vi "ADIS16448 IMU Example.vi"() -> ()   [LabVIEW 2015]
doc: "SimpleGyro Example\n\nThis example shows how to use a SimpleGyro sensor connected to the SPI port on the RoboRIO.\n\nThis example expects a USB cable connected from your development PC to the Type B USB Jack (next to the power input) on the roboRIO."
uses:
  <vilib>/Rock Robotics/SystemInterfaces/spilib/spi_bus.ctl
  ADI MXP IMU/FRC_ADIS16448_IMU.lvlib
panel:
  out "IMU Angle Delta":cluster{"X":dbl, "Y":dbl, "Z":dbl} {"X" scale=-180.0..180.0; "Y" scale=-180.0..180.0; "Z" scale=-180.0..180.0}
  out "IMU AHRS":cluster{"Pitch":dbl, "Roll":dbl, "Yaw":dbl} {"Roll" scale=-180.0..180.0; "Pitch" scale=-90.0..90.0}
  out "IMU Data Out":T1 {"X Accel (g)" format="%#_3g"; "Y Accel (g)" format="%#_3g"; "Z Accel (g)" format="%#_3g"}
  in  "AHRS Algorithm":enum16{"Complementary", "Madgwick"}(ring)
  in  "AHRS Yaw Axis":enum16{"X", "Y", "Z"}(ring)=enum."Z"
  out "Sensor Ready?":bool
  out "IMU AHRS":cluster{"Pitch":dbl, "Roll":dbl, "Yaw":dbl}
  out "IMU Angle Delta":cluster{"X":dbl, "Y":dbl, "Z":dbl}
  in  "Reset Deltas?":bool
  out "Device Found?":bool
  in  "stop":bool
  # "FRC Analog Devices ADIS16448 IMU Example"
  # "Raw IMU Output Data"
  # "FRC ADI MXP Placement"
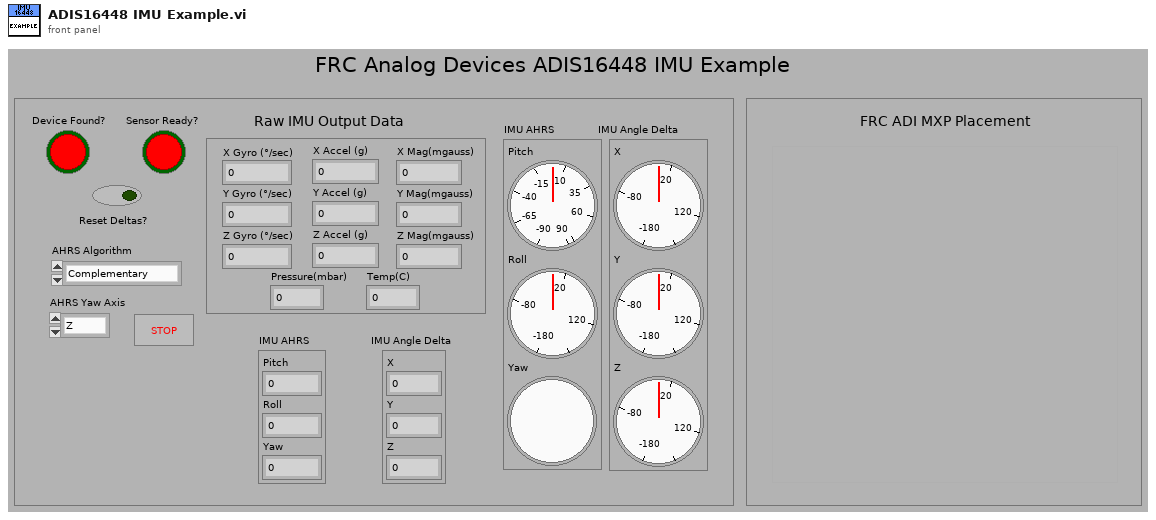
[diagram p1: front panel]
types:
  T1 = cluster{"X Gyro (°/sec)":dbl, "Y Gyro (°/sec)":dbl, "Z Gyro (°/sec)":dbl, "X Accel (g)":dbl, "Y Accel (g)":dbl, "Z Accel (g)":dbl, "X Mag(mgauss)":dbl, "Y Mag(mgauss)":dbl, "Z Mag(mgauss)":dbl, "Pressure(mbar)":dbl, "Temp(C)":dbl}
  T2 = typedef "spi_bus.ctl" = enum16{"SPI On-Board, CS0", "SPI On-Board, CS1", "SPI On-Board, CS2", "SPI On-Board, CS3", "SPI MXP", "Invalid"}
  T3 = typedef "FRC_ADIS16448_IMU.lvlib/WPI_IMU_ADIS16448_InterruptDevRef.ctl" = cluster{"ADI IMU DevRef":T4, "InterruptRef":T5}
  T4 = typedef "FRC_ADIS16448_IMU.lvlib/WPI_IMU_ADIS16448_IMUDevRef.ctl" = cluster{"DevStatus":errorcluster, "Handle":i32, "SPI Bus":T2, "Device Found":bool, "Device Ready":bool, "Yaw Axis":enum16{"X", "Y", "Z"}, "AHRS Algorithm":enum16{"Complementary", "Madgwick"}, "Serial":u16, "Lot ID 2":u16, "Lot ID 1":u16, "Product ID":u16}
  T5 = typedef "WPI_InterruptRef.ctl" = cluster{"DevStatus":errorcluster, "InterruptIndex":T6}
  T6 = typedef "FPGA_InterruptIndex.ctl" = enum8{"0", "1", "2", "3", "4", "5", "6", "7", "Invalid"}
  T7 = cluster{"X Angle":dbl, "Y Angle":dbl, "Z Angle":dbl}
  T8 = cluster{"X Gyro":dbl, "Y Gyro":dbl, "Z Gyro":dbl, "X Accel":dbl, "Y Accel":dbl, "Z Accel":dbl, "X Mag":dbl, "Y Mag":dbl, "Z Mag":dbl, "Pressure":dbl, "Temp":dbl}
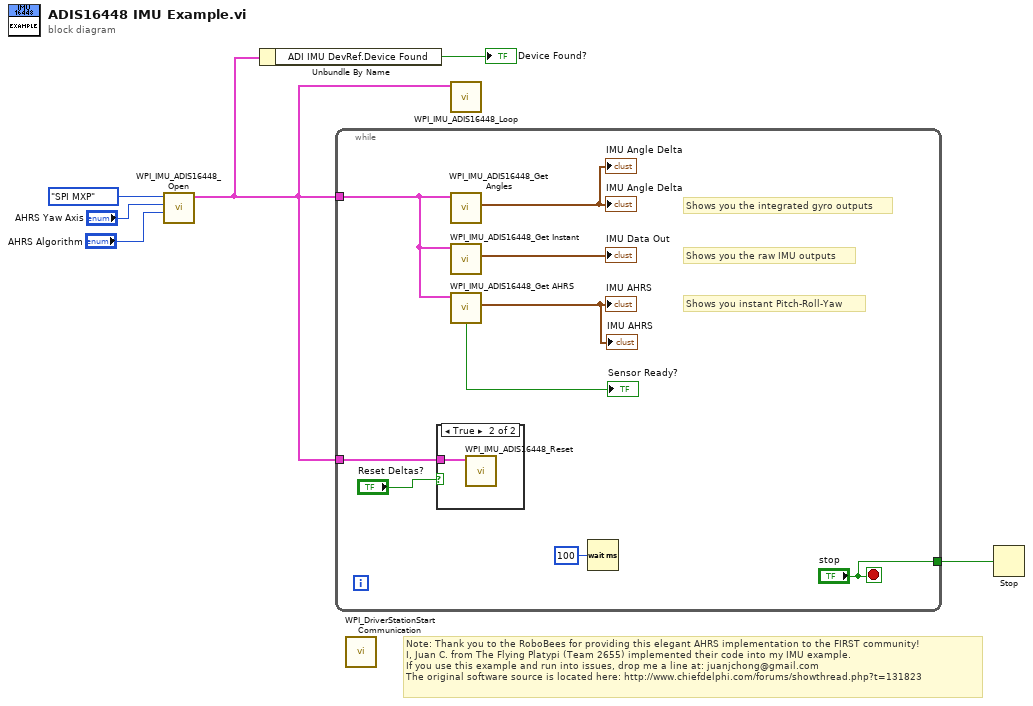
[diagram p0: block diagram]
diagram:
  # "Note: Thank you to the RoboBees for providing this elegant AHRS implementation to the FIRST community!\nI, Juan C. from The Flying Platypi (Team 2655) implemented their code into my IMU example.\nIf you use this example and run into issues, drop me a line at: juanjchong@gmail.com\nThe original software source is located here: http://www.chiefdelphi.com/forums/showthread.php?t=131823"
  n1 = call "WPI_IMU_ADIS16448_Open.vi"("AHRS Algorithm"="AHRS Algorithm", "Yaw Axis"="AHRS Yaw Axis", "SPI Chip Select"=spi_bus."SPI MXP") -> ("ADI IMU Interrupt DevRef"=w1:T3)  [unwired: 7 in, 1 out]
  n2 = Unbundle By Name(w1) -> ("ADI IMU DevRef.Device Found"=→"Device Found?":bool)
  n3 = while {
    tunnel: w1 -> [w11]
    tunnel: ["stop"] -> w5
    tunnel: w1 -> [w14]
    stop <- "stop" stop-if-true
    # "Shows you the integrated gyro outputs"
    # "Shows you the raw IMU outputs"
    # "Shows you instant Pitch-Roll-Yaw"
    n4 = case shown="True" "Reset Deltas?" {
      tunnel: w14 -> [_ w16]
      frame False {
      }
      frame True {
        n5 = call "WPI_IMU_ADIS16448_Reset.vi"("ADI IMU Interrupt DevRef"=w16) -> ()  [unwired: 9 in, 2 out]
      }
    }
    n6 = call "WPI_IMU_ADIS16448_Get Angles.vi"("ADI IMU Interrupt DevRef"=w11) -> ("IMU Angles Out"=→"IMU Angle Delta" →"IMU Angle Delta":T7)  [unwired: 7 in, 3 out]
    n7 = call "WPI_IMU_ADIS16448_Get Instant.vi"("ADI IMU Interrupt DevRef"=w11) -> ("IMU Data Out"=→"IMU Data Out":T8)  [unwired: 7 in, 3 out]
    n8 = call "WPI_IMU_ADIS16448_Get AHRS.vi"("ADI IMU Interrupt DevRef"=w11) -> ("IMU AHRS Out"=→"IMU AHRS" →"IMU AHRS":cluster{"Pitch":dbl, "Roll":dbl, "Yaw":dbl}, "Sensor Ready Out"=→"Sensor Ready?":bool)  [unwired: 6 in, 3 out]
    n9 = Wait (ms)(milliseconds to wait=u32 100) -> ()  [unwired: 1 out]
  }
  n10 = call <vilib>:"WPI_DriverStationStart Communication.vi"() -> ()  [unwired: 12 in]
  n11 = call "WPI_IMU_ADIS16448_Loop.vi"("ADI IMU Interrupt DevRef"=w1) -> ()  [unwired: 9 in, 2 out]
  n12 = Stop(stop? (T)=w5) -> ()
